vi "Controle_Manip_Main_GUI_WorkingBackup_211222.vi"() -> ()   [LabVIEW 2019] (continued)
          n58 = control-ref of="Shutter Ctrls"() -> (w62:refnum<vi>)
          n59 = control-ref of="Save Polarisation"() -> (w56:refnum<vi>)
          n60 = Bundle("Scan Main Progess Bar"=w45, "Acquire XY Map"=w46, "MasterPause"=w31, "MasterStop"=w30, "Save XY Map"=w47, "Scan X Readout (V)"=w48, "Scan Y Readout (V)"=w49, "CCD 1D Spectrum XY Map"=w50, "XY Intensity Map"=w51, "CCD 2D Image XY Map"=w52, "Expected (s)"=w53, "Elapsed (s)"=w54, "Cnts"=w43) -> (→"Scan XY Map References":T31)  [unwired: 1 in]
          n61 = Bundle("Acquire Polarisation"=w55, "Save Polarisation"=w56, "MasterPause"=w33, "MasterStop"=w32, "Scan Main Progess Bar"=w57, "RotStage Exc Angle Readout (°)"=w58, "RotStage Det Angle Readout (°)"=w59, "Polarisation 1D Spectrum"=w60, "Polarisation 2D Image"=w61, "Shutter Ctrls"=w62, "KCube Shutter Device Reference"=w63) -> (→"Scan Polarisation References":T32)  [unwired: 1 in]
          n62 = control-ref of="Contrast Oscillations"() -> (w70:refnum<vi>)
          n63 = control-ref of="Acquire Contrast"() -> (w69:refnum<vi>)
          n64 = control-ref of="Contrast 1D Spectrum"() -> (w71:refnum<vi>)
          n65 = control-ref of="Save Contrast"() -> (w68:refnum<vi>)
          n66 = control-ref of="Att Pos X"() -> (w36:refnum<vi>)
          n67 = control-ref of="Att Pos Y"() -> (w35:refnum<vi>)
          n68 = control-ref of="Att Pos Z"() -> (w37:refnum<vi>)
          n69 = control-ref of="KCube Shutter Device Reference"() -> (w75:refnum<vi>)
          n70 = control-ref of="PZC Position Readout (usteps)"() -> (w74:refnum<vi>)
          n71 = control-ref of="Stop Contrast"() -> (w72:refnum<vi>)
          n72 = control-ref of="Scan Main Progess Bar"() -> (w67:refnum<vi>)
          n73 = control-ref of="Scan Y Readout (V)"() -> (w41:refnum<vi>)
          n74 = control-ref of="Scan X Readout (V)"() -> (w40:refnum<vi>)
          n75 = local write "NewVal"(FALSE ("NewVal")) -> ()
          n76 = control-ref of="Map Marker X Pos"() -> (w39:refnum<vi>)
          n77 = control-ref of="Map Marker Y Pos"() -> (w38:refnum<vi>)
          n78 = control-ref of="Pause Contrast"() -> (w73:refnum<vi>)
          n79 = control-ref of="Shutter Ctrls"() -> (w65:refnum<vi>)
          n80 = Bundle("Shutter Ctrls"=w65, "KCube Shutter Device Reference"=w75, "Scan Main Progess Bar"=w67, "PZC Position Readout (usteps)"=w74, "Pause Contrast"=w73, "Stop Contrast"=w72, "Contrast 1D Spectrum"=w71, "Contrast Oscillations"=w70, "Acquire Contrast"=w69, "Save Contrast"=w68) -> (→"Contrast References":T14)  [unwired: 1 in]
          n81 = Bundle("Scan Y Readout (V)"=w41, "Scan X Readout (V)"=w40, "Map Marker X Pos"=w39, "Map Marker Y Pos"=w38, "Att Pos Z"=w37, "Att Pos X"=w36, "Att Pos Y"=w35) -> (→"Location Parameters":T6)  [unwired: 1 in]
          n82 = local write "Log file"(w76) -> ()
          n83 = local write "Comment"(w76) -> ()
        }
        frame #3 {
          # "Get Experiment Graph Control numbers"
          n84 = control-ref of="Experiment Graph Controls"() -> (w80:refnum<vi>)
          n85 = property class="TabCtl (strict)"(reference=w80) -> ("Pages"=w78:refnum<vi>[])  [unwired: 1 in, 2 out]
          n86 = call "TabVisibility.vi"("Page Visible"=TRUE, "array"=w78, "MyfinalExpGraphCont"=T28."Absorption" ("Experiment Graph Controls")) -> ()  [unwired: 1 in]
        }
      }
    }
    frame #1 {
      # "Initialisation of all the devices?"
      # "Initialisation of devices connections"
      n87 = call "Initialisation prompt"() -> ("Yes please!"=w81:bool)  [unwired: 18 in, 1 out]
      "Initialise all devices?" <- w81
      n88 = case shown="True" w81 {
        frame False {
          # "Do not activate devices"
          n89 = control-ref of="Tab Objective Sample"() -> (w88:refnum<vi>)
          n90 = property on="Experimental parameters tab" class="TabCtl (strict)" props=["Pages", "Value"]() -> ("Pages"=w90:refnum<vi>[])  [unwired: 2 in, 3 out]
          n91 = property class="TabCtl (strict)"(reference=w88) -> ("Pages"=w86:refnum<vi>[])  [unwired: 1 in, 2 out]
          n92 = property on="Experiment Graph Controls" class="TabCtl (strict)" props=["Value", "Pages"]() -> ("Pages"=w92:refnum<vi>[])  [unwired: 2 in, 3 out]
          n93 = Array Size(array=w86) -> (size(s)=w87:i32)
          n94 = Array Size(array=w90) -> (size(s)=w89:i32)
          n95 = for {
            N: w89 -> [_]
            tunnel: w90 -> [w99]
            i -> [w97]
            n96 = Index Array(array=w99, index=w97) -> (element=w100:refnum<vi>)
            n97 = property class="Page"(reference=w100, "PageVis"=TRUE ("Page Visible")) -> ()  [unwired: 1 in, 2 out]
          }
          n98 = for {
            N: w87 -> [_]
            tunnel: w86 -> [w96]
            i -> [w95]
            n99 = Index Array(array=w96, index=w95) -> (element=w94:refnum<vi>)
            n100 = property class="Page"(reference=w94, "PageVis"=TRUE ("Page Visible")) -> ()  [unwired: 1 in, 2 out]
          }
          n101 = Array Size(array=w92) -> (size(s)=w91:i32)
          n102 = for {
            N: w91 -> [_]
            tunnel: w92 -> [w103]
            i -> [w101]
            n103 = Index Array(array=w103, index=w101) -> (element=w104:refnum<vi>)
            n104 = property class="Page"(reference=w104, "PageVis"=TRUE ("Page Visible")) -> ()  [unwired: 1 in, 2 out]
          }
          n105 = local read "Log file"() -> (w84:string)
          n106 = call "Write2LogFile.vi"("Add to log file"="Initialisation ...\nNo instruments activated.", "Log file before"=w84, "Checkbox"=FALSE) -> ("Log file after"=w85:string)
          n107 = local write "Log file"(w85) -> ()
        }
        frame True {
          # "Activate all the devices selected in the Settings tab"
          n108 = stacked-sequence {
            frame #0 {
              n109 = local read "ESP 301 On?"() -> (w113:bool)
              n110 = local read "ESP 300 On?"() -> (w114:bool)
              n111 = local read "PZC200 On?"() -> (w107:bool)
              n112 = local write "Scan Main Progess Bar"(u8 0 ("Scan Main Progess Bar")) -> ()
              n113 = local read "KCube Shutter On?"() -> (w111:bool)
              n114 = local read "KCubes Piezo On?"() -> (w110:bool)
              n115 = local read "Laser Comm On?"() -> (w105:bool)
              n116 = local read "Cryostation On?"() -> (w115:bool)
              n117 = local read "Attocubes On?"() -> (w116:bool)
              n118 = local read "PM16-120 On?"() -> (w108:bool)
              n119 = local read "LightField On?"() -> (w109:bool)
              n120 = local read "PicoHarp On?"() -> (w106:bool)
              n121 = local read "FSM 300 On?"() -> (w112:bool)
              n122 = global write "InstrumentsOn.vi" "ESP 301 On?"(w113) -> ()
              n123 = global write "InstrumentsOn.vi" "ESP 300 On?"(w114) -> ()
              n124 = global write "InstrumentsOn.vi" "PZC200 On?"(w107) -> ()
              n125 = global write "InstrumentsOn.vi" "Attocubes On?"(w116) -> ()
              n126 = global write "InstrumentsOn.vi" "Cryostation On?"(w115) -> ()
              n127 = global write "InstrumentsOn.vi" "PM16-120 On?"(w108) -> ()
              n128 = global write "InstrumentsOn.vi" "LightField On?"(w109) -> ()
              n129 = global write "InstrumentsOn.vi" "Laser Comm On?"(w105) -> ()
              n130 = global write "InstrumentsOn.vi" "KCubes Piezo On?"(w110) -> ()
              n131 = global write "InstrumentsOn.vi" "KCube Shutter On?"(w111) -> ()
              n132 = global write "InstrumentsOn.vi" "FSM 300 On?"(w112) -> ()
              n133 = global write "InstrumentsOn.vi" "PicoHarp On?"(w106) -> ()
            }
            frame #1 {
              # "LLTF"
              n134 = case shown="True" "LLTF On?" {
                frame False {
                }
                frame True {
                  n135 = Automation Open(Automation Refnum="xphyspecLib.IXPhySpec") -> (Automation Refnum=w136:refnum<k7>, error out=w135:errorcluster)  [unwired: 3 in]
                  n136 = local read "Excitation Wavelength (nm)"() -> (w126:dbl)
                  n137 = call "newinit.vi"("error in"=w135, "Automation Refnum"=w136) -> ("error out"=w132:errorcluster, "Detected?"=→"LLTF Detected?":bool, "xphyspecLib.IXPhySpec out"=w133:refnum<k7>)  [unwired: 7 in]
                  n138 = call "listandgetdeviceinterface.vi"("error in (no error)"=w132, "reference"=w133) -> ("LLTF error out"=→"LLTFDevice error out":errorcluster, "LLTFDevice Interface"=w128:refnum<k7>, "error out to close"=→"LLTF Error":errorcluster, "reference out to lose"=→"LLTF Reference":refnum<k7>)  [unwired: 6 in]
                  n139 = call "testmove.vi"("p_TargetWavelength"=w126, "reference"=w128) -> ("CurrentWavelength"=→"CurrentWL":dbl, "CurrentAngle"=→"CurrentAngle":dbl, "Device reference out"=→"LLTFDevice Interface":refnum<k7>, "Device moved"=→"Device moved":bool)  [unwired: 4 in, 2 out]
                  n140 = local read "Log file"() -> (w122:string)
                  n141 = call "Write2LogFile.vi"("Add to log file"="Initialise communication with PhotonEtc LLTF", "Log file before"=w122, "Checkbox"=FALSE) -> ("Log file after"=w121:string)
                  n142 = local write "Log file"(w121) -> ()
                }
              }
            }
            frame #2 {
              # "ESP 300: 1 Jobin Yvon 320 Monochromator"
              n143 = control-ref of="CCD 1D Spectrum Main  Cursor2WL 1 Mono 2"() -> (w140:refnum<vi>)
              n144 = control-ref of="CCD 1D Spectrum Main  Cursor2WL 2 Mono 2"() -> (w139:refnum<vi>)
              n145 = local read "ESP300 COM Port"() -> (w138:refnum<visa-resource-name>)
              n146 = case shown="True" "ESP 300 On?" {
                tunnel: [enum16{"Enabled", "Disabled", "Disabled&Grayed"}."Disabled&Grayed" ("Enum") enum16{"Enabled", "Disabled", "Disabled&Grayed"}."Enabled" ("Enum")] -> w142
                tunnel: w138 -> [w147 w150]
                frame False {
                  n147 = global write "InstrumentReferences.vi" "ESP300 COM Port"(w147) -> ()
                }
                frame True {
                  n148 = global write "InstrumentReferences.vi" "ESP300 COM Port"(w150) -> ()
                  n149 = control-ref of="Mono2 Velocity"() -> (w154:refnum<vi>)
                  n150 = control-ref of="Mono2 Motor Pos"() -> (w153:refnum<vi>)
                  n151 = call "subVI_Init&GetParams.vi"("Mono2 Pos"=w153, "Mono2 Velocity"=w154) -> ("Mono2 On"=w155:bool)  [unwired: 1 in]
                  n152 = local read "Log file"() -> (w159:string)
                  n153 = local write "Mono2 On"(w155) -> ()
                  n154 = call "Write2LogFile.vi"("Add to log file"="Initialise communication with ESP 300", "Log file before"=w159, "Checkbox"=FALSE) -> ("Log file after"=w158:string)
                  n155 = local write "Log file"(w158) -> ()
                  n156 = control-ref of="Mono2 Wavelength (nm)"() -> (w152:refnum<vi>)
                  n157 = property class="DigNum (strict)"(reference=w152, "DisabledEnum"=T29."Disabled and Grayed Out" ("Disabled")) -> ()  [unwired: 1 in, 2 out]
                }
              }
              n158 = control-ref of="Mono2 On"() -> (w143:refnum<vi>)
              n159 = control-ref of="Mono2 Wavelength (nm)"() -> (w144:refnum<vi>)
              n160 = control-ref of="Mono2 Motor Pos"() -> (w141:refnum<vi>)
              n161 = Build Array(w143, w144, w141, w140, w139) -> (w145:refnum<vi>[])
              n162 = call "Enable&Disable_Controls.vi"("Enum"=w142, "References"=w145) -> ()  [unwired: 1 in]
            }
            frame #3 {
              # "ESP 301: 2 rotation stages + 1 linear translation stage"
              n163 = case shown="True" "ESP 301 On?" {
                frame False {
                  n164 = control-ref of="Experiment Graph Controls"() -> (w163:refnum<vi>)
                  n165 = local read "Scan Polar AllParams"() -> (w175:refnum<vi>[])
                  n166 = property class="TabCtl (strict)"(reference=w163) -> ("Pages"=w167:refnum<vi>[])  [unwired: 1 in, 2 out]
                  n167 = property class="TabCtl (strict)"(reference=w163) -> ("Pages"=w164:refnum<vi>[])  [unwired: 1 in, 2 out]
                  n168 = call "Enable&Disable_Controls.vi"("Enum"=enum16{"Enabled", "Disabled", "Disabled&Grayed"}."Disabled&Grayed", "References"=w175) -> ()  [unwired: 1 in]
                  n169 = property on="Experimental parameters tab" class="TabCtl (strict)"() -> ("Pages"=w170:refnum<vi>[])  [unwired: 2 in, 2 out]
                  n170 = call "TabVisibility.vi"("Page Visible"=FALSE, "array"=w167, "MyfinalExpGraphCont"=T28."Polarisation Acquisition") -> ()  [unwired: 1 in]
                  n171 = call "TabVisibility.vi"("Page Visible"=FALSE, "array"=w164, "MyfinalExpGraphCont"=T28."Contrast Acquisition") -> ()  [unwired: 1 in]
                  n172 = local read "Scan Translation Coarse Ctrls"() -> (w169:refnum<vi>[])
                  n173 = Index Array(array=w170, index=2) -> (element=w177:refnum<vi>)
                  n174 = Index Array(array=w170, index=3) -> (element=w171:refnum<vi>)
                  n175 = property class="Page"(reference=w171, "PageVis"=FALSE ("Page Visible")) -> ()  [unwired: 1 in, 2 out]
                  n176 = property class="Page"(reference=w177, "PageVis"=FALSE ("Page Visible")) -> ()  [unwired: 1 in, 2 out]
                  n177 = call "Enable&Disable_Controls.vi"("Enum"=enum16{"Enabled", "Disabled", "Disabled&Grayed"}."Disabled&Grayed", "References"=w169) -> ()  [unwired: 1 in]
                }
                frame True {
                  n178 = stacked-sequence {
                    frame #0 {
                      n179 = local read "Log file"() -> (w182:string)
                      n180 = call "Write2LogFile.vi"("Add to log file"="Initialise communication with ESP 301", "Log file before"=w182, "Checkbox"=FALSE) -> ("Log file after"=w180:string)
                      n181 = local write "Log file"(w180) -> ()
                    }
                    frame #1 {
                      n182 = control-ref of="Experiment Graph Controls"() -> (w189:refnum<vi>)
                      n183 = property class="TabCtl (strict)"(reference=w189) -> ("Pages"=w190:refnum<vi>[])  [unwired: 1 in, 2 out]
                      n184 = property on="Experimental parameters tab" class="TabCtl (strict)"("Value"=T19."Polarisation" ("Experimental parameters tab")) -> ("Pages"=w195:refnum<vi>[])  [unwired: 2 in, 2 out]
                      n185 = property on="Experimental parameters tab" class="TabCtl (strict)"() -> ("Pages"=w202:refnum<vi>[])  [unwired: 2 in, 2 out]
                      n186 = property class="TabCtl (strict)"(reference=w189) -> ("Pages"=w193:refnum<vi>[])  [unwired: 1 in, 2 out]
                      n187 = call "TabVisibility.vi"("Page Visible"=TRUE, "array"=w190, "MyfinalExpGraphCont"=T28."Contrast Acquisition") -> ()  [unwired: 1 in]
                      n188 = Index Array(array=w195, index=3) -> (element=w198:refnum<vi>)
                      n189 = Index Array(array=w202, index=2) -> (element=w199:refnum<vi>)
                      n190 = call "TabVisibility.vi"("Page Visible"=TRUE, "array"=w193, "MyfinalExpGraphCont"=T28."Polarisation Acquisition") -> ()  [unwired: 1 in]
                      n191 = property class="Page"(reference=w199, "PageVis"=TRUE ("Page Visible")) -> ()  [unwired: 1 in, 2 out]
                      n192 = property class="Page"(reference=w198, "PageVis"=TRUE ("Page Visible")) -> ()  [unwired: 1 in, 2 out]
                      n193 = local read "Scan Translation Coarse Ctrls"() -> (w188:refnum<vi>[])
                      n194 = local read "Scan Polar AllParams"() -> (w186:refnum<vi>[])
                      n195 = call "Enable&Disable_Controls.vi"("Enum"=enum16{"Enabled", "Disabled", "Disabled&Grayed"}."Enabled", "References"=w188) -> ()  [unwired: 1 in]
                      n196 = call "Enable&Disable_Controls.vi"("Enum"=enum16{"Enabled", "Disabled", "Disabled&Grayed"}."Enabled", "References"=w186) -> ()  [unwired: 1 in]
                    }
                    frame #2 {
                      n197 = flat-sequence {
                        tunnel: [w209] -> w203
                        frame #0 {
                          w209 = refnum<visa-resource-name> "COM8" ("ESP 301 COM Port")
                          n198 = call "Close.vi"("VISA resource name"=w209) -> ()  [unwired: 10 in, 1 out]
                        }
                        frame #1 {
                          n199 = call "_Create Instrument Channel_libESP301.vi"("COM Port (1)"=u16 8) -> ()  [unwired: 8 in, 3 out]
                        }
                      }
                      n200 = call "Initialize.vi"("VISA resource name"=w203, "ID Query (True)"=TRUE, "Reset (False)"=FALSE ("ID Query (True)"), "Serial Link (RS232)"=enum16{"RS232", "USB"}."USB") -> ("VISA resource name out"=w204:refnum<visa-resource-name>, "error out"=w208:errorcluster)  [unwired: 5 in]
                      n201 = case shown="Default" w208 {
                        tunnel: w204 -> [_ _]
                        frame No Error {
                        }
                        frame Default {
                          w216 = FALSE ("ID Query (True)")
                          n202 = call "Connect Newport Instruments_libESP301.vi"() -> ("error (duplicate)"=w214:errorcluster, "VISA resource name (duplicate)"=w211:refnum<visa-resource-name>)  [unwired: 7 in, 3 out]
                          n203 = call "_Close Communications_libESP301.vi"("Instrument Channel"=w211, "error in (no error)"=w214) -> ("error out"=w213:errorcluster)  [unwired: 13 in]
                          n204 = call "Initialize.vi"("VISA resource name"=w211, "ID Query (True)"=w216, "Reset (False)"=w216, "error in (no error)"=w213, "Serial Link (RS232)"=enum16{"RS232", "USB"}."USB") -> ("VISA resource name out"=w212:refnum<visa-resource-name>)  [unwired: 4 in, 1 out]
                          n205 = local write "ESP 301 COM Port"(w212) -> ()
                        }
                      }
                      n206 = local write "ESP 301 COM Port"(w204) -> ()
                    }
                    frame #3 {
                      # "Initialise ESP301 communication\nand motor parameters & limits"
                      n207 = local read "ESP 301 COM Port"() -> (w217:refnum<visa-resource-name>)
                      n208 = for {
                        N: 3 -> [_]
                        tunnel: w217 -> [w230]
                        tunnel: [w229] -> _
                        i -> [w220]
                        n209 = Increment(x=w220) -> (x+1=w219:i32)
                        n210 = call "Get Left Travel Limit.vi"("Axis (1)"=w219, "VISA resource name"=w230) -> ("Left Travel Limit (units)"=w226:dbl, "VISA resource name out"=w233:refnum<visa-resource-name>)  [unwired: 3 in, 1 out]
                        n211 = call "Get Right Travel Limit.vi"("Axis (1)"=w219, "VISA resource name"=w233) -> ("Right Travel Limit (units)"=w225:dbl, "VISA resource name out"=w232:refnum<visa-resource-name>)  [unwired: 3 in, 1 out]
                        n212 = call "Get Velocity.vi"("Axis (1)"=w219, "VISA resource name"=w232) -> ("Velocity (units/s)"=w224:dbl, "VISA resource name out"=w231:refnum<visa-resource-name>)  [unwired: 3 in, 1 out]
                        n213 = call "Read Actual Position.vi"("Axis (1)"=w219, "VISA resource name"=w231) -> ("Position (units)"=w221:dbl, "VISA resource name out"=w228:refnum<visa-resource-name>)  [unwired: 3 in, 1 out]
                        n214 = call "Get Maximum Velocity.vi"("Axis (1)"=w219, "VISA resource name"=w228) -> ("Maximum Velocity (units/s)"=w223:dbl, "VISA resource name out"=w227:refnum<visa-resource-name>)  [unwired: 3 in, 1 out]
                        n215 = call "Get Motor Power Status.vi"("Axis (1)"=w219, "VISA resource name"=w227) -> ("Power Status"=w222:bool, "VISA resource name out"=w229:refnum<visa-resource-name>)  [unwired: 3 in, 1 out]
                        n216 = case shown="1" w219 {
                          tunnel: w226 -> [_ w239 w245 w251]
                          tunnel: w225 -> [_ w238 w244 w250]
                          tunnel: w224 -> [_ w237 w243 w248]
                          tunnel: w223 -> [_ w236 w241 w249]
                          tunnel: w222 -> [_ w235 w240 w246]
                          tunnel: w221 -> [_ w234 w242 w247]
                          frame 0, Default {
                          }
                          frame 1 {
                            # "Translation stage"
                            n217 = property on="Newport Linear Translation Stage Position (mm)" class="DigNum (strict)"("Minimum"=w239, "Maximum"=w238) -> ()  [unwired: 2 in, 2 out]
                            n218 = local write "Newport Linear Translation Stage Velocity (mm/s)"(w237) -> ()
                            n219 = local write "Newport Linear Translation Stage Position Readout (mm)"(w234) -> ()
                            n220 = property on="Newport Linear Translation Stage Velocity (mm/s)" class="DigNum (strict)"("Maximum"=w236) -> ()  [unwired: 2 in, 2 out]
                            n221 = local write "Motor LinT On?"(w235) -> ()
                          }
                          frame 2 {
                            # "RotStage Det"
                            n222 = property on="RotStage Det Angle (°)" class="DigNum (strict)"("Maximum"=w245, "Minimum"=w244) -> ()  [unwired: 2 in, 2 out]
                            n223 = local write "RotStage Det Velocity (°/s)"(w243) -> ()
                            n224 = property on="RotStage Det Velocity (°/s)" class="DigNum (strict)"("Maximum"=w241) -> ()  [unwired: 2 in, 2 out]
                            n225 = local write "RotStage Det Angle Readout (°)"(w242) -> ()
                            n226 = local write "Motor RotStage Det On?"(w240) -> ()
                          }
                          frame 3 {
                            # "RotStage Exc"
                            n227 = property on="RotStage Exc Angle (°)" class="DigNum (strict)"("Maximum"=w251, "Minimum"=w250) -> ()  [unwired: 2 in, 2 out]
                            n228 = local write "RotStage Exc Velocity (°/s)"(w248) -> ()
                            n229 = property on="RotStage Exc Velocity (°/s)" class="DigNum (strict)"("Maximum"=w249) -> ()  [unwired: 2 in, 2 out]
                            n230 = local write "RotStage Exc Angle Readout (°)"(w247) -> ()
                            n231 = local write "Motor RotStage Exc On?"(w246) -> ()
                          }
                        }
                      }
                    }
                    frame #4 {
                      n232 = local read "ESP 301 COM Port"() -> (w252:refnum<visa-resource-name>)
                      n233 = call "Get Motor Power Status.vi"("Axis (1)"=1, "VISA resource name"=w252) -> ("error out"=w259:errorcluster, "Power Status"=w255:bool, "VISA resource name out"=w260:refnum<visa-resource-name>)  [unwired: 3 in]
                      n234 = local write "Motor LinT On?"(w255) -> ()
                      n235 = call "Get Motor Power Status.vi"("error in (no error)"=w259, "Axis (1)"=2, "VISA resource name"=w260) -> ("error out"=w262:errorcluster, "Power Status"=w253:bool, "VISA resource name out"=w261:refnum<visa-resource-name>)  [unwired: 2 in]
                      n236 = local write "Motor RotStage Exc On?"(w253) -> ()
                      n237 = call "Get Motor Power Status.vi"("error in (no error)"=w262, "Axis (1)"=3, "VISA resource name"=w261) -> ("error out"=w263:errorcluster, "Power Status"=w254:bool)  [unwired: 2 in, 1 out]
                      n238 = local write "Motor RotStage Det On?"(w254) -> ()
                      n239 = local write "ESP 301 Error"(w263) -> ()
                    }
                  }
                }
              }
            }
            frame #4 {
              # "Advance progress bar"
              n240 = local write "Scan Main Progess Bar"(u8 5 ("Scan Main Progess Bar")) -> ()
            }
            frame #5 {
              # "LightField: Monochromator SpectraPro HRS-500 + CCD Pixis"
              n241 = case shown="True" "LightField On?" {
                frame False {
                  n242 = control-ref of="Grating"() -> (w279:refnum<vi>)
                  n243 = control-ref of="Center Wavelength (nm)"() -> (w281:refnum<vi>)
                  n244 = local read "PicoHarp On?"() -> (w287:bool)
                  n245 = local read "ESP 300 On?"() -> (w288:bool)
                  n246 = control-ref of="Accumulations"() -> (w284:refnum<vi>)
                  n247 = control-ref of="CCD ROI"() -> (w283:refnum<vi>)
                  n248 = control-ref of="Exposure Time (ms)"() -> (w282:refnum<vi>)
                  n249 = control-ref of="Exit mirror"() -> (w280:refnum<vi>)
                  n250 = And(x=w288, y=w287) -> (x .and. y?=w286:bool)
                  n251 = case shown="False" w286 {
                    frame False {
                      n252 = control-ref of="Experiment Graph Controls"() -> (w290:refnum<vi>)
                      n253 = property class="TabCtl (strict)"(reference=w290) -> ("Pages"=w292:refnum<vi>[])  [unwired: 1 in, 2 out]
                      n254 = call "TabVisibility.vi"("Page Visible"=FALSE, "array"=w292, "MyfinalExpGraphCont"=T28."Spectrum Acquisition") -> ()  [unwired: 1 in]
                    }
                    frame True {
                      n255 = control-ref of="Experiment Graph Controls"() -> (w294:refnum<vi>)
                      n256 = property class="TabCtl (strict)"(reference=w294) -> ("Pages"=w296:refnum<vi>[])  [unwired: 1 in, 2 out]
                      n257 = call "TabVisibility.vi"("Page Visible"=TRUE, "array"=w296, "MyfinalExpGraphCont"=T28."Spectrum Acquisition") -> ()  [unwired: 1 in]
                    }
                  }
                  n258 = Build Array(w281, w280, w279, w284, w283, w282) -> (w285:refnum<vi>[])
                  n259 = call "Enable&Disable_Controls.vi"("Enum"=enum16{"Enabled", "Disabled", "Disabled&Grayed"}."Disabled&Grayed", "References"=w285) -> ()  [unwired: 1 in]
                  n260 = control-ref of="Experiment Graph Controls"() -> (w277:refnum<vi>)
                  n261 = control-ref of="Experiment Graph Controls"() -> (w272:refnum<vi>)
                  n262 = control-ref of="Experiment Graph Controls"() -> (w271:refnum<vi>)
                  n263 = property class="TabCtl (strict)"(reference=w277) -> ("Pages"=w275:refnum<vi>[])  [unwired: 1 in, 2 out]
                  n264 = property class="TabCtl (strict)"(reference=w272) -> ("Pages"=w274:refnum<vi>[])  [unwired: 1 in, 2 out]
                  n265 = property class="TabCtl (strict)"(reference=w271) -> ("Pages"=w269:refnum<vi>[])  [unwired: 1 in, 2 out]
                  n266 = call "TabVisibility.vi"("Page Visible"=FALSE, "array"=w275, "MyfinalExpGraphCont"=T28."Intensity Map Acquisition") -> ()  [unwired: 1 in]
                  n267 = call "TabVisibility.vi"("Page Visible"=FALSE, "array"=w274, "MyfinalExpGraphCont"=T28."Polarisation Acquisition") -> ()  [unwired: 1 in]
                  n268 = call "TabVisibility.vi"("Page Visible"=FALSE, "array"=w269, "MyfinalExpGraphCont"=T28."Contrast Acquisition") -> ()  [unwired: 1 in]
                }
                frame True {
                  n269 = stacked-sequence {
                    seq-local: [_ _ "uPL" ("ExperimentName") _ _ _ _] -> [_ _ _ w327 _ _ _]
                    seq-local: [_ _ w321 _ _ _ _] -> [_ _ _ w328 _ _ _]
                    seq-local: [_ _ w320 _ _ _ _] -> [_ _ _ w326 _ _ _]
                    seq-local: [_ _ _ w325 _ _ _] -> [_ _ _ _ w337 _ _]
                    seq-local: [_ _ _ w324 _ _ _] -> [_ _ _ _ w336 _ _]
                    seq-local: [_ _ _ _ w331 _ _] -> [_ _ _ _ _ w344 _]
                    seq-local: [_ _ _ _ w332 _ _] -> [_ _ _ _ _ w345 _]
                    seq-local: [_ _ _ _ w330 _ _] -> [_ _ _ _ _ w343 _]
                    frame #0 {
                      n270 = control-ref of="Grating"() -> (w299:refnum<vi>)
                      n271 = control-ref of="Center Wavelength (nm)"() -> (w301:refnum<vi>)
                      n272 = control-ref of="Accumulations"() -> (w304:refnum<vi>)
                      n273 = control-ref of="CCD ROI"() -> (w303:refnum<vi>)
                      n274 = control-ref of="Exposure Time (ms)"() -> (w302:refnum<vi>)
                      n275 = control-ref of="Exit mirror"() -> (w300:refnum<vi>)
                      n276 = local read "Log file"() -> (w307:string)
                      n277 = Build Array(w301, w300, w299, w304, w303, w302) -> (w305:refnum<vi>[])
                      n278 = call "Write2LogFile.vi"("Add to log file"="Launching LightField (~ 20 s)", "Log file before"=w307, "Checkbox"=FALSE) -> ("Log file after"=w308:string)
                      n279 = call "Enable&Disable_Controls.vi"("Enum"=enum16{"Enabled", "Disabled", "Disabled&Grayed"}."Enabled", "References"=w305) -> ()  [unwired: 1 in]
                      n280 = local write "Log file"(w308) -> ()
                    }
                    frame #1 {
                      n281 = control-ref of="Experiment Graph Controls"() -> (w310:refnum<vi>)
                      n282 = control-ref of="Experimental parameters tab"() -> (w314:refnum<vi>)
                      n283 = property class="TabCtl (strict)"(reference=w310) -> ("Pages"=w312:refnum<vi>[])  [unwired: 1 in, 2 out]
                      n284 = property class="TabCtl (strict)"(reference=w314, "Value"=T19."Monochromators & CCD") -> ("Pages"=w317:refnum<vi>[])  [unwired: 1 in, 2 out]
                      n285 = call "TabVisibility.vi"("Page Visible"=TRUE, "array"=w312, "MyfinalExpGraphCont"=T28."Spectrum Acquisition") -> ()  [unwired: 1 in]
                      n286 = Index Array(array=w317, index=0) -> (element=w318:refnum<vi>)
                      n287 = property class="Page"(reference=w318, "PageVis"=TRUE ("Page Visible")) -> ()  [unwired: 1 in, 2 out]
                    }
                    frame #2 {
                      n288 = call "LFA_Initialize.vi"("Is Visible?"="LF Visible") -> ("error out"=w321:errorcluster, "LightField Automation out"=w320:refnum<class "LightField Automation.lvclass">)  [unwired: 9 in]
                    }
                    frame #3 {
                      n289 = local write "Scan Main Progess Bar"(u8 15 ("Scan Main Progess Bar")) -> ()
                      n290 = call "Exp_SetExperiment.vi"("error in (no error)"=w328, "ExperimentName"=w327, "LightField Automation in"=w326) -> ("error out"=w325:errorcluster, "LightField Automation out"=w324:refnum<class "LightField Automation.lvclass">)  [unwired: 7 in]
                    }
                    frame #4 {
                      n291 = local read "Log file"() -> (w335:string)
                      n292 = call "Write2LogFile.vi"("Add to log file"="Getting parameters", "Log file before"=w335, "Checkbox"=FALSE) -> ("Log file after"=w334:string)
                      n293 = local write "Log file"(w334) -> ()
                      n294 = call "Exp_CCD_GetExposureTime.vi"("error in (no error)"=w337, "LightField Automation in"=w336) -> ("error out"=w331:errorcluster, "Exposure Time (s)"=w330:dbl, "LightField Automation out"=w332:refnum<class "LightField Automation.lvclass">)  [unwired: 7 in]
                    }
                    frame #5 {
                      n295 = call "Exp_CCD_GetTemperature.vi"("error in (no error)"=w344, "LightField Automation in"=w345) -> ("error out"=w348:errorcluster, "Temperature (°C)"=→"CCD T° :":dbl, "LightField Automation out"=w347:refnum<class "LightField Automation.lvclass">)  [unwired: 7 in]
                      n296 = call "spec_GetGratings.vi"("error in (no error)"=w348, "LightField Automation in"=w347) -> ("error out"=w356:errorcluster, "Current Grating"=w350:string, "LightField Automation out"=w357:refnum<class "LightField Automation.lvclass">)  [unwired: 6 in, 1 out]
                      n297 = call "spec_GetCenterWavelength.vi"("error in (no error)"=w356, "LightField Automation in"=w357) -> ("error out"=w354:errorcluster, "Center Wavelength"=w351:dbl, "LightField Automation out"=w353:refnum<class "LightField Automation.lvclass">)  [unwired: 7 in]
                      n298 = local write "Grating"(w350) -> ()
                      n299 = call "spec_getCalibration.vi"("error in (no error)"=w354, "LightField Automation in"=w353) -> ("error out"=w341:errorcluster, "ColumnCalibration"=→"Wavelength calibration":dbl[], "LightField Automation out"=w342:refnum<class "LightField Automation.lvclass">)  [unwired: 7 in]
                      n300 = call "spec_GetOpticalExitPort.vi"("error in (no error)"=w341, "LightField Automation in"=w342) -> ("error out"=w340:errorcluster, "Exit Port Location"=w339:T33, "LightField Automation out"=w338:refnum<class "LightField Automation.lvclass">)  [unwired: 7 in]
                      n301 = local write "Center Wavelength (nm)"(w351) -> ()
                      n302 = global write "InstrumentReferences.vi" "LightField Automation out"(w338) -> ()
                      n303 = local write "LightField Automation out"(w338) -> ()
                      n304 = local write "LightField Automation error out"(w340) -> ()
                      n305 = local write "Exit mirror"(w339) -> ()
                      n306 = Multiply(x=w343, y=1000.0) -> (x*y=w352:dbl)
                      n307 = local write "Exposure Time (ms)"(w352) -> ()
                      n308 = local write "Acq Time (ms)"(w352) -> ()
                    }
                    frame #6 {
                      n309 = local write "Scan Main Progess Bar"(u8 35 ("Scan Main Progess Bar")) -> ()
                    }
                  }
                }
              }
            }
            frame #6 {
              # "Thorlabs USB photodiode"
              n310 = case shown="True" "PM16-120 On?" {
                frame False {
                  n311 = property on="Excitation Power (uW)" class="DigNum (strict)"("Label.BG Color"=u32 16711680 ("Label.Colors:BG Color")) -> ()  [unwired: 2 in, 2 out]
                }
                frame True {
                  w362 = refnum<visa-resource-name> "USB0::0x1313::0x807B::190927109::INSTR" ("instrument handle")
                  # "Initialise powermeter"
                  n312 = call <instrlib>:"TLPM Find Resources.vi"("instrument handle"=w362) -> ("error out"=w367:errorcluster, "Resource Count"=w369:u32)  [unwired: 8 in, 1 out]
                  n313 = property on="Excitation Power (uW)" class="DigNum (strict)"("Blinking"=FALSE) -> ()  [unwired: 2 in, 2 out]
                  n314 = Greater Or Equal?(x=w369, y=1) -> (x >= y?=w368:bool)
                  n315 = case shown="True" w368 {
                    tunnel: w367 -> [_ w382]
                    tunnel: w362 -> [w374 w375]
                    frame False {
                      w373 = FALSE ("ID Query (Do Query)")
                      n316 = call <instrlib>:"TLPM Initialize.vi"("Reset Device (Reset Device)"=w373, "ID Query (Do Query)"=w373, "resource name"=w374) -> ("error out"=w371:errorcluster, "instrument handle out"=w372:refnum<visa-resource-name>)  [unwired: 7 in]
                      n317 = local write "Photodiode handle out"(w372) -> ()
                      n318 = local write "Photodiode error out"(w371) -> ()
                    }
                    frame True {
                      w381 = FALSE ("Reset Device (Reset Device)")
                      # "Select first Device\n(Device Index 0)"
                      n319 = call <instrlib>:"TLPM Get Resource Name.vi"("error in (no error)"=w382, "Index (0)"=u32 0) -> ("error out"=w380:errorcluster)  [unwired: 7 in, 2 out]
                      n320 = local write "Photodiode Status"(TRUE) -> ()
                      n321 = call <instrlib>:"TLPM Initialize.vi"("error in (no error)"=w380, "Reset Device (Reset Device)"=w381, "ID Query (Do Query)"=w381, "resource name"=w375) -> ("error out"=w377:errorcluster, "instrument handle out"=w378:refnum<visa-resource-name>)  [unwired: 6 in]
                      n322 = local write "Photodiode handle out"(w378) -> ()
                      n323 = local write "Photodiode error out"(w377) -> ()
                    }
                  }
                  n324 = local read "Log file"() -> (w366:string)
                  n325 = call "Write2LogFile.vi"("Add to log file"="Initialise communication with Photodiode", "Log file before"=w366, "Checkbox"=FALSE) -> ("Log file after"=w365:string)
                  n326 = local write "Log file"(w365) -> ()
                }
              }
            }
            frame #7 {
              # "448.3nm Laser Diode + Temp Controller & Driver"
              n327 = case shown="True" "Laser Comm On?" {
                frame False {
                  w384 = FALSE ("Visible")
                  n328 = property on="TEC Output" class="Bool (strict)"("Visible"=w384) -> ()  [unwired: 2 in, 2 out]
                  n329 = property on="TEC Temperature" class="DigNum (strict)"("Visible"=w384) -> ()  [unwired: 2 in, 2 out]
                  n330 = property on="Laser Diode Current Set" class="Slide (strict)"("Visible"=w384) -> ()  [unwired: 2 in, 2 out]
                  n331 = property on="Laser on? Control" class="Bool (strict)"("Visible"=w384) -> ()  [unwired: 2 in, 2 out]
                }
                frame True {
                  n332 = local read "Log file"() -> (w388:string)
                  n333 = call "Write2LogFile.vi"("Add to log file"="Initialise communication with Laser Driver", "Log file before"=w388, "Checkbox"=FALSE) -> ("Log file after"=w387:string)
                  n334 = local write "Log file"(w387) -> ()
                  n335 = call "LaserDiodeInit.vi"("resource name"=refnum<visa-resource-name> "USB0::0x1313::0x804F::M00549740::INSTR" ("Diode Driver COM")) -> ("Diode Driver Error"=w393:errorcluster, "Temperature"=w390:dbl, "TEC Output"=w392:bool, "resource out"=→"DDE":refnum<visa-resource-name>, "LD Output"=w391:bool, "Serial Number"=→"Serial Number":string)
                  n336 = local write "Laser on?"(w391) -> ()
                  n337 = local write "Laser on? Control"(w391) -> ()
                  n338 = local write "TEC Output"(w392) -> ()
                  n339 = local write "TEC Temperature"(w390) -> ()
                  n340 = local write "Diode Driver Error"(w393) -> ()
                  n341 = property on="Laser Diode Current Set" class="Slide (strict)"("Visible"=w392) -> ()  [unwired: 2 in, 2 out]
                  n342 = property on="Laser Safety" class="Ring (strict)"("Visible"=w392) -> ()  [unwired: 2 in, 2 out]
                  n343 = property on="Laser on? Control" class="Bool (strict)"("Visible"=w392) -> ()  [unwired: 2 in, 2 out]
                }
              }
            }
            frame #8 {
              # "Excitation wavelength"
              n344 = disable-structure shown="Enabled" {
                disable-tunnel: [w399 458.3] -> w398
                frame Disabled {
                  n345 = call "PromptUserWavelength_DefautValue.vi"() -> ("Wavelength"=w399:dbl)  [unwired: 17 in, 2 out]
                }
                frame Enabled {
                }
              }
              n346 = call "nm2WL.vi"("Wavelength (380 - 780)"=w398) -> ("Color"=w396:u32, "Out Of Range"=w397:bool)
              n347 = case shown="False" w397 {
                tunnel: w396 -> [w404 _]
                frame False {
                  # "set laser color"
                  n348 = Bundle("Color"=w404, "Color"=w404) -> (w403:cluster{"Color":u32, "Color":u32})  [unwired: 1 in]
                  n349 = Bundle(u32 16777216, u32 16777216) -> (w402:cluster{u32, u32})  [unwired: 1 in]
                  n350 = Build Array(w402, w403) -> (w401:cluster{"Color":u32, "Color":u32}[])
                  n351 = property on="Laser on?" class="Bool (strict)"("Colors [4]"=w401) -> ()  [unwired: 2 in, 2 out]
                }
                frame True {
                }
              }
              n352 = local write "Excitation Wavelength (nm)"(w398) -> ()
            }
            frame #9 {
              # "Advancec progress bar"
              n353 = local write "Scan Main Progess Bar"(u8 50 ("Scan Main Progess Bar")) -> ()
            }
            frame #10 {
              # "FSM"
              n354 = local read "FSM 300 On?"() -> (w408:bool)
              n355 = case shown="True" w408 {
                frame True {
                  n356 = stacked-sequence {
                    frame #0 {
                      n357 = local read "Log file"() -> (w412:string)
                      n358 = call "Write2LogFile.vi"("Add to log file"="Initialise communication with FSM", "Log file before"=w412, "Checkbox"=FALSE) -> ("Log file after"=w411:string)
                      n359 = local write "Log file"(w411) -> ()
                    }
                    frame #1 {
                      n360 = control-ref of="Experiment Graph Controls"() -> (w413:refnum<vi>)
                      n361 = property on="Experimental parameters tab" class="TabCtl (strict)"("Value"=T19."Steering mirror" ("Experimental parameters tab")) -> ("Pages"=w421:refnum<vi>[])  [unwired: 2 in, 2 out]
                      n362 = property class="TabCtl (strict)"(reference=w413) -> ("Pages"=w415:refnum<vi>[])  [unwired: 1 in, 2 out]
                      n363 = Index Array(array=w421, index=1) -> (element=w419:refnum<vi>)
                      n364 = property class="Page"(reference=w419, "PageVis"=TRUE ("Page Visible")) -> ()  [unwired: 1 in, 2 out]
                      n365 = call "TabVisibility.vi"("Page Visible"=TRUE, "array"=w415, "MyfinalExpGraphCont"=T28."Intensity Map Acquisition" ("Experiment Graph Controls")) -> ()  [unwired: 1 in]
                    }
                    frame #2 {
                      w426 = 10.0 ("maximum value")
                      w428 = 10.0 ("maximum value")
                      n366 = local read "FSM Y Axis"() -> (w424:tag)
                      n367 = local read "FSM X Axis"() -> (w427:tag)
                      n368 = Negate(x=w428) -> (-x=w429:dbl)
                      n369 = Negate(x=w426) -> (-x=w425:dbl)
                      n370 = call-poly <vilib>:"DAQmx Create Virtual Channel.vi"("maximum value"=w428, "minimum value"=w429, "physical channels"=w427) -> ("task out"=→"FSM X Task":refnum<k21>)  [unwired: 11 in, 1 out]
                      n371 = call-poly <vilib>:"DAQmx Create Virtual Channel.vi"("maximum value"=w426, "minimum value"=w425, "physical channels"=w424) -> ("task out"=→"FSM Y Task":refnum<k21>)  [unwired: 11 in, 1 out]
                    }
                  }
                }
                frame False {
                  n372 = control-ref of="Experiment Graph Controls"() -> (w431:refnum<vi>)
                  n373 = property on="Experimental parameters tab" class="TabCtl (strict)"() -> ("Pages"=w437:refnum<vi>[])  [unwired: 2 in, 2 out]
                  n374 = property class="TabCtl (strict)"(reference=w431) -> ("Pages"=w433:refnum<vi>[])  [unwired: 1 in, 2 out]
                  n375 = Index Array(array=w437, index=1) -> (element=w435:refnum<vi>)
                  n376 = call "TabVisibility.vi"("Page Visible"=FALSE, "array"=w433, "MyfinalExpGraphCont"=T28."Intensity Map Acquisition") -> ()  [unwired: 1 in]
                  n377 = property class="Page"(reference=w435, "PageVis"=FALSE ("Page Visible")) -> ()  [unwired: 1 in, 2 out]
                }
              }
            }
            frame #11 {
              # "Set all graph styles according to CCD Acq Mode: Spectrum or 2D Image"
              n378 = local read "Acq Mode"() -> (w438:T3)
              n379 = case shown="\"Image\"" w438 {
                frame "Image" {
                  w460 = TRUE
                  w459 = FALSE
                  n380 = property on="CCD 2D Image Main" class="IntGraph (strict)"("Visible"=w460) -> ()  [unwired: 2 in, 2 out]
                  n381 = property on="CCD 2D Image XY Map" class="IntGraph (strict)"("Visible"=w460) -> ()  [unwired: 2 in, 2 out]
                  n382 = property on="CCD 1D Spectrum XY Map" class="WFGraph (strict)"("Visible"=w459) -> ()  [unwired: 2 in, 2 out]
                  n383 = property on="CCD 1D Spectrum Main" class="XYGraph (strict)"("Visible"=w459) -> ()  [unwired: 2 in, 2 out]
                }
                frame "Spectrum" {
                  w461 = FALSE
                  w462 = TRUE
                  n384 = property on="CCD 2D Image Main" class="IntGraph (strict)"("Visible"=w461) -> ()  [unwired: 2 in, 2 out]
                  n385 = property on="CCD 2D Image XY Map" class="IntGraph (strict)"("Visible"=w461) -> ()  [unwired: 2 in, 2 out]
                  n386 = property on="CCD 1D Spectrum XY Map" class="WFGraph (strict)"("Visible"=w462) -> ()  [unwired: 2 in, 2 out]
                  n387 = property on="CCD 1D Spectrum Main" class="XYGraph (strict)"("Visible"=w462) -> ()  [unwired: 2 in, 2 out]
                }
                frame "APD 1" {
                  w463 = FALSE
                  w464 = TRUE
                  n388 = property on="CCD 2D Image Main" class="IntGraph (strict)"("Visible"=w463) -> ()  [unwired: 2 in, 2 out]
                  n389 = property on="CCD 2D Image XY Map" class="IntGraph (strict)"("Visible"=w463) -> ()  [unwired: 2 in, 2 out]
                  n390 = property on="CCD 1D Spectrum XY Map" class="WFGraph (strict)"("Visible"=w464) -> ()  [unwired: 2 in, 2 out]
                  n391 = property on="CCD 1D Spectrum Main" class="XYGraph (strict)"("Visible"=w464) -> ()  [unwired: 2 in, 2 out]
                }
                frame "APD 2" {
                  w465 = FALSE
                  w466 = TRUE
                  n392 = property on="CCD 2D Image Main" class="IntGraph (strict)"("Visible"=w465) -> ()  [unwired: 2 in, 2 out]
                  n393 = property on="CCD 2D Image XY Map" class="IntGraph (strict)"("Visible"=w465) -> ()  [unwired: 2 in, 2 out]
                  n394 = property on="CCD 1D Spectrum XY Map" class="WFGraph (strict)"("Visible"=w466) -> ()  [unwired: 2 in, 2 out]
                  n395 = property on="CCD 1D Spectrum Main" class="XYGraph (strict)"("Visible"=w466) -> ()  [unwired: 2 in, 2 out]
                }
                frame "APD 1+2" {
                  w467 = FALSE
                  w468 = TRUE
                  n396 = property on="CCD 2D Image Main" class="IntGraph (strict)"("Visible"=w467) -> ()  [unwired: 2 in, 2 out]
                  n397 = property on="CCD 2D Image XY Map" class="IntGraph (strict)"("Visible"=w467) -> ()  [unwired: 2 in, 2 out]
                  n398 = property on="CCD 1D Spectrum XY Map" class="WFGraph (strict)"("Visible"=w468) -> ()  [unwired: 2 in, 2 out]
                  n399 = property on="CCD 1D Spectrum Main" class="XYGraph (strict)"("Visible"=w468) -> ()  [unwired: 2 in, 2 out]
                }
              }
              n400 = case shown="\"Spectrum\", Default" w438 {
                frame "Image" {
                  n401 = control-ref of="Experiment Graph Controls"() -> (w441:refnum<vi>)
                  n402 = property class="TabCtl (strict)"(reference=w441) -> ("Pages"=w442:refnum<vi>[])  [unwired: 1 in, 2 out]
                  n403 = call "TabVisibility.vi"("Page Visible"=FALSE, "array"=w442, "MyfinalExpGraphCont"=T28."Spectrum Acquisition") -> ()  [unwired: 1 in]
                }
                frame "Spectrum", Default {
                  n404 = control-ref of="Experiment Graph Controls"() -> (w444:refnum<vi>)
                  n405 = property class="TabCtl (strict)"(reference=w444) -> ("Pages"=w446:refnum<vi>[])  [unwired: 1 in, 2 out]
                  n406 = call "TabVisibility.vi"("Page Visible"=FALSE, "array"=w446, "MyfinalExpGraphCont"=T28."APDs Acquisition") -> ()  [unwired: 1 in]
                }
                frame "APD 1" {
                  n407 = control-ref of="Experiment Graph Controls"() -> (w448:refnum<vi>)
                  n408 = property class="TabCtl (strict)"(reference=w448) -> ("Pages"=w450:refnum<vi>[])  [unwired: 1 in, 2 out]
                  n409 = call "TabVisibility.vi"("Page Visible"=TRUE, "array"=w450, "MyfinalExpGraphCont"=T28."APDs Acquisition") -> ()  [unwired: 1 in]
                }
                frame "APD 2" {
                  n410 = control-ref of="Experiment Graph Controls"() -> (w452:refnum<vi>)
                  n411 = property class="TabCtl (strict)"(reference=w452) -> ("Pages"=w454:refnum<vi>[])  [unwired: 1 in, 2 out]
                  n412 = call "TabVisibility.vi"("Page Visible"=TRUE, "array"=w454, "MyfinalExpGraphCont"=T28."APDs Acquisition") -> ()  [unwired: 1 in]
                }
                frame "APD 1+2" {
                  n413 = control-ref of="Experiment Graph Controls"() -> (w456:refnum<vi>)
                  n414 = property class="TabCtl (strict)"(reference=w456) -> ("Pages"=w458:refnum<vi>[])  [unwired: 1 in, 2 out]
                  n415 = call "TabVisibility.vi"("Page Visible"=TRUE, "array"=w458, "MyfinalExpGraphCont"=T28."APDs Acquisition") -> ()  [unwired: 1 in]
                }
              }
            }
            frame #12 {
              # "KCubes: 1 Shutter + 3 Piezos for XYZ microscope objective"
              n416 = stacked-sequence {
                frame #0 {
                  # "Shutter"
                  n417 = case shown="True" "KCube Shutter On?" {
                    frame False {
                      n418 = control-ref of="Experimental parameters tab"() -> (w474:refnum<vi>)
                      n419 = property class="TabCtl (strict)"(reference=w474) -> ("Pages"=w472:refnum<vi>[])  [unwired: 1 in, 2 out]
                      n420 = Index Array(array=w472, index=5) -> (element=w471:refnum<vi>)
                      n421 = property class="Page"(reference=w471, "PageVis"=FALSE ("Page Visible")) -> ()  [unwired: 1 in, 2 out]
                    }
                    frame True {
                      n422 = stacked-sequence {
                        frame #0 {
                          n423 = local read "Log file"() -> (w478:string)
                          n424 = call "Write2LogFile.vi"("Add to log file"="Initialise communication with Shutter", "Log file before"=w478, "Checkbox"=FALSE) -> ("Log file after"=w477:string)
                          n425 = local write "Log file"(w477) -> ()
                        }
                        frame #1 {
                          n426 = control-ref of="Experimental parameters tab"() -> (w484:refnum<vi>)
                          n427 = property class="TabCtl (strict)"(reference=w484, "Value"=T19."Shutter options") -> ("Pages"=w482:refnum<vi>[])  [unwired: 1 in, 2 out]
                          n428 = Index Array(array=w482, index=5) -> (element=w481:refnum<vi>)
                          n429 = property class="Page"(reference=w481, "PageVis"=TRUE ("Page Visible")) -> ()  [unwired: 1 in, 2 out]
                        }
                        frame #2 {
                          n430 = Wait (ms)(milliseconds to wait=u32 50) -> ()  [unwired: 1 out]
                        }
                        frame #3 {
                          n431 = local read "KCubeSolenoidControl"() -> (w487:refnum<k24>)
                          n432 = property class="KCubeSolenoidControl"(reference=w487, "SerialNumber"="68001425") -> (reference out=w488:refnum<k24>)  [unwired: 1 in, 1 out]
                          n433 = invoke class="KCubeSolenoidControl" method="CreateDevice"(reference=w488) -> (reference out=w489:refnum<k24>)  [unwired: 2 in, 2 out]
                          n434 = property class="KCubeSolenoidControl"(reference=w489) -> (reference out=w490:refnum<k24>, "Device"=w491:refnum<k24>)  [unwired: 1 in, 1 out]
                          n435 = invoke class="KCubeSolenoid" method="GetOperatingState"(reference=w491) -> (reference out=w492:refnum<k24>, "GetOperatingState"=w493:i32)  [unwired: 2 in, 1 out]
                          n436 = local write "KCubeSolenoidControl Reference"(w490) -> ()
                          n437 = case shown="2, Default" w493 {
                            frame 1 {
                              n438 = property on="Shutter Ctrls" class="Ring (strict)"("Value"=u16 5 ("Shutter Ctrls")) -> ()  [unwired: 2 in, 2 out]
                            }
                            frame 2, Default {
                              n439 = property on="Shutter Ctrls" class="Ring (strict)"("Value"=u16 0 ("Shutter Ctrls")) -> ()  [unwired: 2 in, 2 out]
                            }
                          }
                          n440 = local write "KCube Shutter Device Reference"(w492) -> ()
                        }
                      }
                    }
                  }
                }
                frame #1 {
                  # "Piezos objective"
                  n441 = case shown="True" "KCubes Piezo On?" {
                    tunnel: [FALSE ("Page Visible") TRUE] -> w497
                    frame False {
                      n442 = disable-structure shown="Disabled" {
                        frame Disabled {
                          n443 = control-ref of="Experimental parameters tab"() -> (w503:refnum<vi>)
                          n444 = property class="TabCtl (strict)"(reference=w503) -> ("Pages"=w506:refnum<vi>[])  [unwired: 1 in, 2 out]
                          n445 = Index Array(array=w506, index=4) -> (element=w507:refnum<vi>)
                          n446 = property class="Page"(reference=w507, "PageVis"=FALSE ("Page Visible")) -> ()  [unwired: 1 in, 2 out]
                        }
                        frame Enabled {
                        }
                      }
                    }
                    frame True {
                      n447 = stacked-sequence {
                        frame #0 {
                          n448 = local read "Log file"() -> (w511:string)
                          n449 = call "Write2LogFile.vi"("Add to log file"="Initialise communication with Objective Piezos", "Log file before"=w511, "Checkbox"=FALSE) -> ("Log file after"=w512:string)
                          n450 = local write "Log file"(w512) -> ()
                        }
                        frame #1 {
                          n451 = control-ref of="Experimental parameters tab"() -> (w516:refnum<vi>)
                          n452 = property class="TabCtl (strict)"(reference=w516, "Value"=T19."Microscope objective") -> ("Pages"=w517:refnum<vi>[])  [unwired: 1 in, 2 out]
                          n453 = Index Array(array=w517, index=4) -> (element=w518:refnum<vi>)
                          n454 = property class="Page"(reference=w518, "PageVis"=TRUE ("Page Visible")) -> ()  [unwired: 1 in, 2 out]
                        }
                        frame #2 {
                          n455 = local read "KCubePiezoControl X"() -> (w524:refnum<k24>)
                          n456 = property class="KCubePiezoControl"(reference=w524, "SerialNumber"="29502682") -> (reference out=w523:refnum<k24>)  [unwired: 1 in, 1 out]
                          n457 = invoke class="KCubePiezoControl" method="CreateDevice"(reference=w523) -> (reference out=w522:refnum<k24>)  [unwired: 2 in, 2 out]
                          n458 = property class="KCubePiezoControl"(reference=w522) -> (reference out=w521:refnum<k24>, "Device"=w520:refnum<k24>)  [unwired: 1 in, 1 out]
                          n459 = local write "KCubePiezoControl X Reference"(w521) -> ()
                          n460 = local write "KCubePiezoDevice X Reference"(w520) -> ()
                        }
                        frame #3 {
                          n461 = local read "KCubePiezoControl Y"() -> (w525:refnum<k24>)
                          n462 = property class="KCubePiezoControl"(reference=w525, "SerialNumber"="29502721") -> (reference out=w527:refnum<k24>)  [unwired: 1 in, 1 out]
                          n463 = invoke class="KCubePiezoControl" method="CreateDevice"(reference=w527) -> (reference out=w528:refnum<k24>)  [unwired: 2 in, 2 out]
                          n464 = property class="KCubePiezoControl"(reference=w528) -> (reference out=w529:refnum<k24>, "Device"=w530:refnum<k24>)  [unwired: 1 in, 1 out]
                          n465 = local write "KCubePiezoControl Y Reference"(w529) -> ()
                          n466 = local write "KCubePiezoDevice Y Reference"(w530) -> ()
                        }
                        frame #4 {
                          n467 = local read "KCubePiezoControl Z"() -> (w532:refnum<k24>)
                          n468 = property class="KCubePiezoControl"(reference=w532, "SerialNumber"="29250034") -> (reference out=w533:refnum<k24>)  [unwired: 1 in, 1 out]
                          n469 = invoke class="KCubePiezoControl" method="CreateDevice"(reference=w533) -> (reference out=w534:refnum<k24>)  [unwired: 2 in, 2 out]
                          n470 = property class="KCubePiezoControl"(reference=w534) -> (reference out=w535:refnum<k24>, "Device"=w536:refnum<k24>)  [unwired: 1 in, 1 out]
                          n471 = local write "KCubePiezoControl Z Reference"(w535) -> ()
                          n472 = local write "KCubePiezoDevice Z Reference"(w536) -> ()
                        }
                        frame #5 {
                          n473 = local read "KCubePiezoDevice Z Reference"() -> (w540:refnum<k24>)
                          n474 = call "KCube_IsActiveAndActivate.vi"("KCubePiezoDevice Z Reference"=w540) -> ("IsSetOutputVoltageActive"=→"IsSetOutputVoltageActive":bool, "reference out"=w538:refnum<k24>, "GetOutputVoltage"=→"GetOutputVoltage":dbl)  [unwired: 8 in]
                          n475 = local write "KCubePiezoDevice Z Reference"(w538) -> ()
                        }
                      }
                    }
                  }
                  n476 = control-ref of="Tab Objective Sample"() -> (w500:refnum<vi>)
                  n477 = property class="TabCtl (strict)"(reference=w500) -> ("Pages"=w499:refnum<vi>[])  [unwired: 1 in, 2 out]
                  n478 = Index Array(array=w499, index=0) -> (element=w498:refnum<vi>)
                  n479 = property class="Page"(reference=w498, "PageVis"=w497) -> ()  [unwired: 1 in, 2 out]
                }
              }
            }
            frame #13 {
              # "Advance progress bar"
              n480 = local write "Scan Main Progess Bar"(u8 70 ("Scan Main Progess Bar")) -> ()
            }
            frame #14 {
              # "PZA12 Fine Delay Translation Stage"
              n481 = case shown="True" "PZC200 On?" {
                frame False {
                  n482 = local read "Scan Contrast Ctrls"() -> (w544:refnum<vi>[])
                  n483 = local read "ESP 301 On?"() -> (w543:bool)
                  n484 = call "Enable&Disable_Controls.vi"("Enum"=enum16{"Enabled", "Disabled", "Disabled&Grayed"}."Disabled&Grayed", "References"=w544) -> ()  [unwired: 1 in]
                  n485 = case shown="True" w543 {
                    frame True {
                      n486 = property on="Experimental parameters tab" class="TabCtl (strict)" props=["Pages", "Value"]() -> ("Pages"=w549:refnum<vi>[])  [unwired: 2 in, 3 out]
                      n487 = property on="Experiment Graph Controls" class="TabCtl (strict)" props=["Value", "Pages"]() -> ("Pages"=w550:refnum<vi>[])  [unwired: 2 in, 3 out]
                      n488 = Index Array(array=w549, index=3) -> (element=w548:refnum<vi>)
                      n489 = Index Array(array=w550, index=3) -> (element=w552:refnum<vi>)